vi "Host.vi"() -> ()   [LabVIEW 2019]
uses:
  <vilib>/Analysis/7linalg.llb/Eigenvalue and Vectors Output Option.ctl
  <vilib>/Analysis/baseanly.llb/Matrix Type of Inverse Matrix.ctl
  <vilib>/Analysis/7linalg.llb/Real Generalized Eigenvalues and Vectors.vi
  <vilib>/Analysis/7linalg.llb/Real Cholesky Factorization.vi
  <vilib>/Analysis/baseanly.llb/Full Cholesky Factorization.vi
  <vilib>/Analysis/baseanly.llb/Full Real Matrix Cholesky Factorization.vi
  <vilib>/FPGAPlugInAG/PXIe-7915/niLvFpga_Open_PXIe-7915.vi
  <vilib>/rvi/interface/common/dynamic/niFpgaDynamicAddResources.vi
  <vilib>/Analysis/baseanly.llb/Real Inverse Matrix.vi
  <vilib>/Analysis/Matrix/Numeric/Multiply/Multiply - RM,RM.vi
  <vilib>/Analysis/7linalg.llb/Real Eigenvalues and Vectors.vi
  <vilib>/Analysis/Matrix/Numeric/Add/Add - RM,RM.vi
  <vilib>/Utility/error.llb/Error Cluster From Error Code.vi
  <vilib>/rvi/errors/niLvFpgaAdjustHostInterfaceError.vi
  <vilib>/FPGAPlugInAG/Dynamic/niLvFpga_Run_Dynamic.vi
  <vilib>/FPGAPlugInAG/Dynamic/niLvFpga_Close_Dynamic.vi
  <vilib>/rvi/interface/nirviOpenFPGA/nirviOpenFPGA.xnode
  FPGA Bitfiles/choleskyfpgav1_FPGATarget_Target_zgTmfM5OUWw.lvbitx
  <vilib>/rvi/interface/nirviMethod/nirviMethod.xnode
  <vilib>/rvi/interface/nirviReadWriteControl/nirviReadWriteControl.xnode
  <vilib>/rvi/interface/nirviCloseFPGA/nirviCloseFPGA.xnode
  <vilib>/Analysis/NI_AALPro.lvlib
  <vilib>/Analysis/NI_AALBase.lvlib
  <vilib>/Analysis/Matrix/NI_Matrix.lvlib
  <vilib>/rvi/errors/niLvFpgaMergeErrorWithErrorCode.vi
  <vilib>/FPGAPlugInAG/Dynamic/niLvFpga_ReadFifo_Dynamic.vi
  <vilib>/FPGAPlugInAG/Dynamic/niLvFpga_WriteFifo_Dynamic.vi
  NiFpgaLv.dll
  <vilib>/rvi/interface/Simulation/niFpgaSimulationCallBeginRW.vi
panel:
  out "total time us":u32
  out "T2 tick (ticks)":u32
  out "T5-T4 us":u32
  out "T4-T3 us":u32
  out "T3-T2 us":u32
  out "T2-T1 us":u32
  out "T5 us":u16
  out "T4 us":u16
  out "T3 us":u16
  out "T2 us":u16
  out "T1 us":u16
  out "data output time (ticks)":u32
  out "data input time (ticks)":u32
  out "total time (ticks)":u32
  out "T5 (ticks)":u32
  out "T4 (ticks)":u32
  out "T3 (ticks)":u32
  out "T1 (ticks)":u32
  out "Frequencies":dbl[](array[numeric])
  out "Eigenvalues":cdb[][](array[numeric]) format="%#_4g"
  out "Run Time (ms)":u32 format="%_6f"
  out "Elements Remaining 2":u32
  out "Elements Remaining":u32
  out "K input":dbl[][](array[numeric])
  in  "Method":i32(listbox)
  out "M input":dbl[][](array[numeric])
  # "Takes 56 ms to solve without timed loop"
  # "base"
  # "1087"
  # "2174"
  # "1087"
  # "97"
  # "1087"
  # "1183"
  # "eith timed loops"
  # "AVG. of 13"
  # "AVG. of 289"
  # "AVG. of 289"
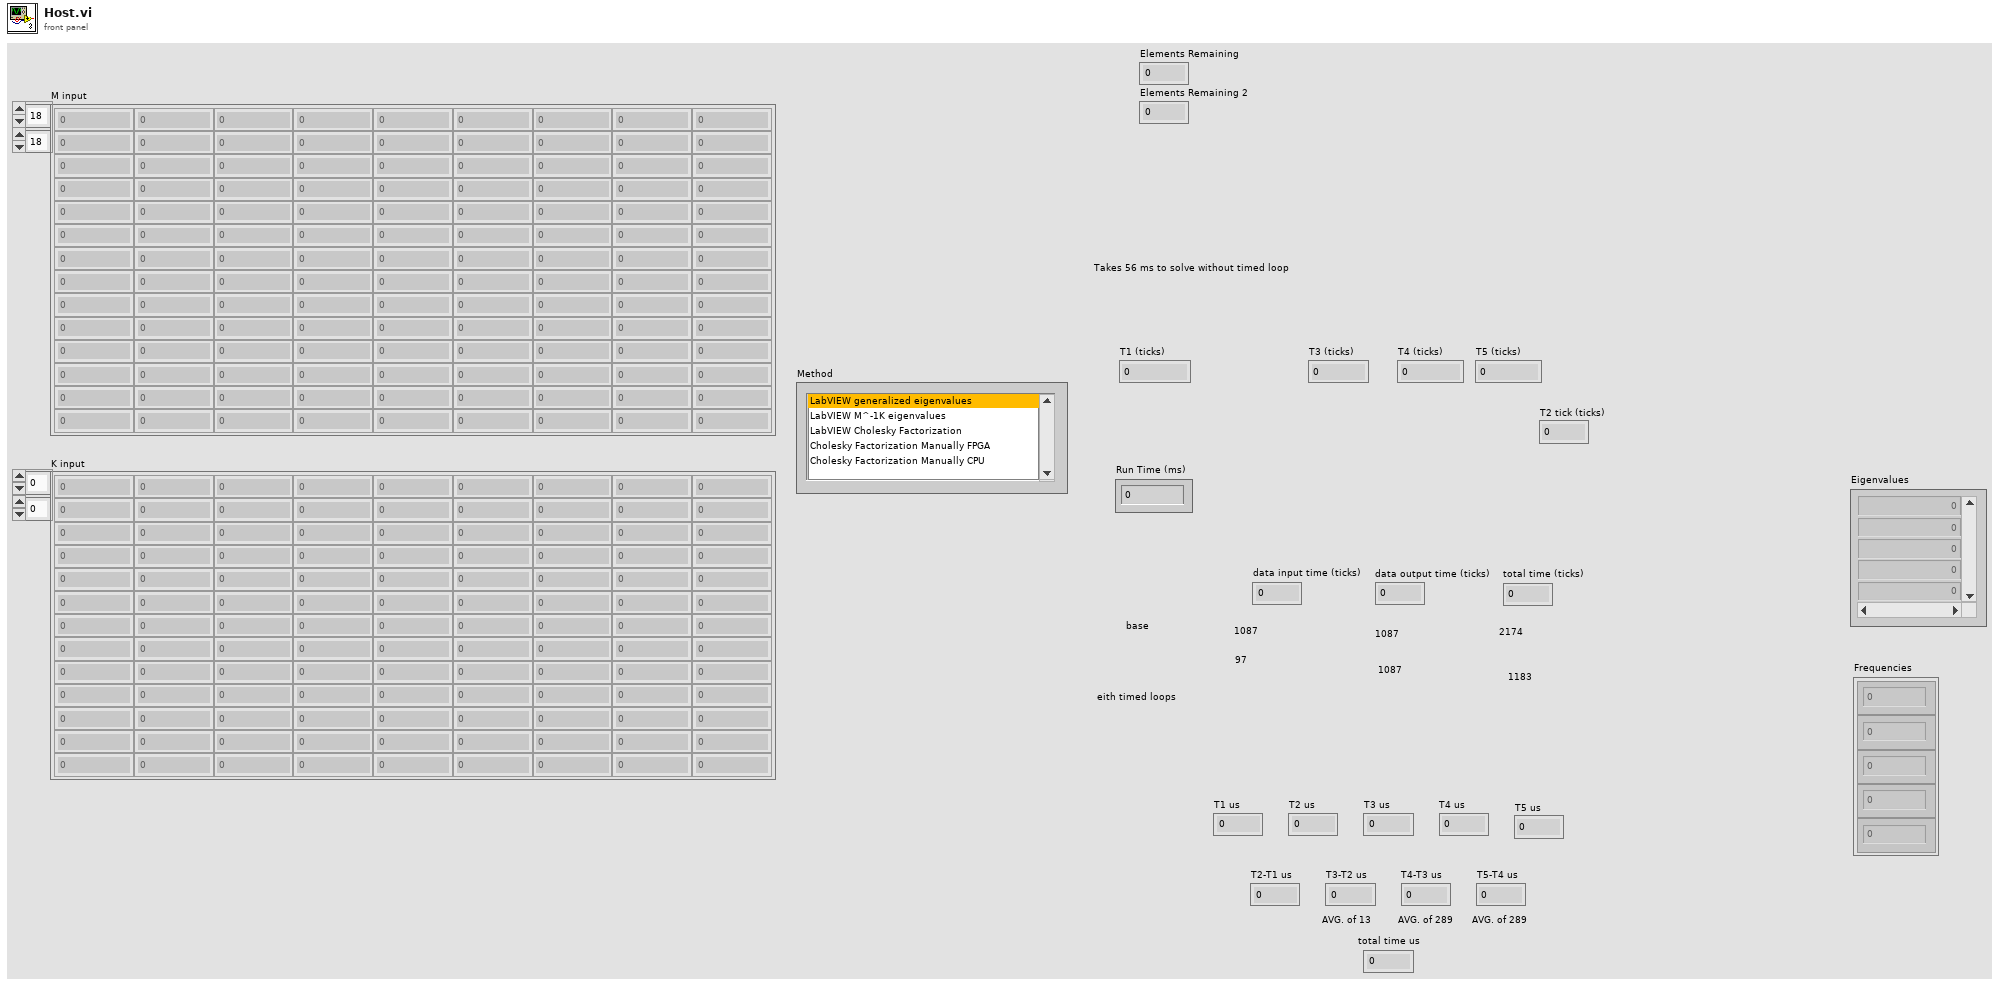
[diagram p1: front panel]
types:
  T1 = typedef "NI_AALBase.lvlib/Matrix Type of Inverse Matrix.ctl" = enum32{"General", "Positive Definite", "Lower Triangular", "Upper Triangular"}
  T2 = typedef "NI_AALPro.lvlib/Eigenvalue and Vectors Output Option.ctl" = i32
  T3 = typedef "NI_Matrix.lvlib/RealMatrix.ctl" = dbl[][]
  T4 = typedef "NI_Matrix.lvlib/ComplexMatrix.ctl" = cdb[][]
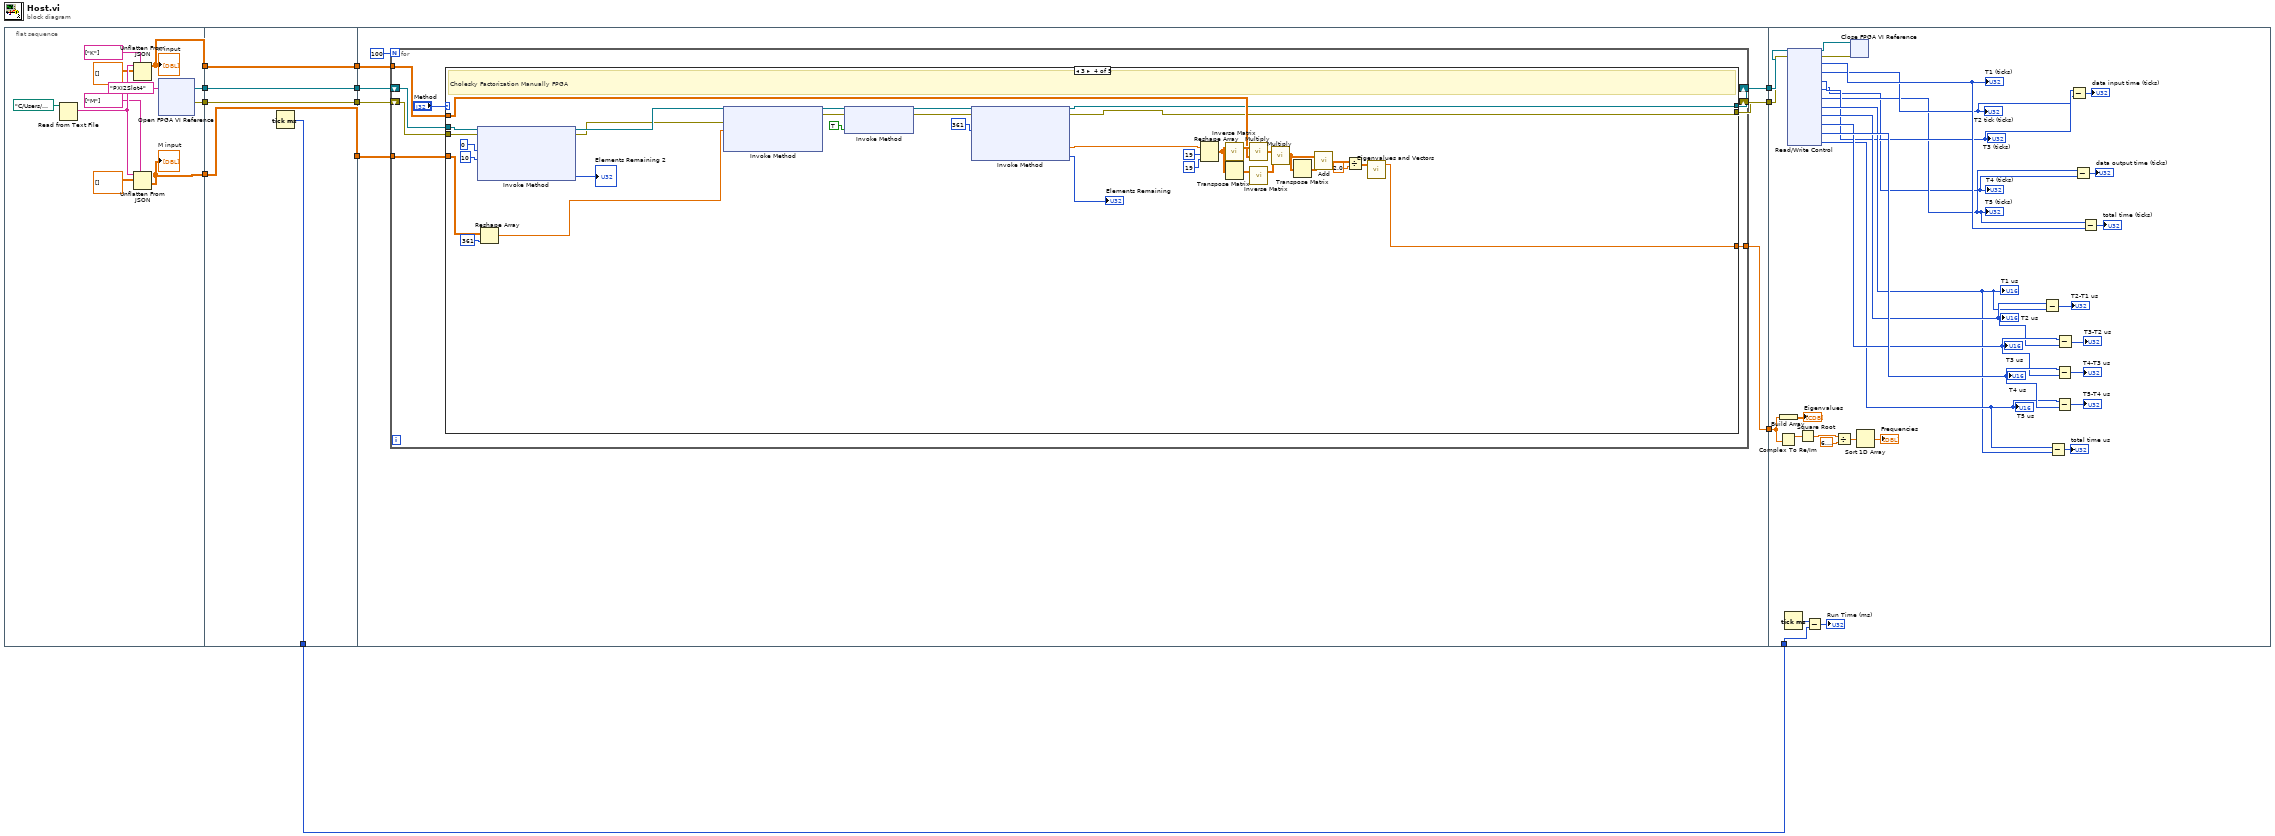
[diagram p0: block diagram]
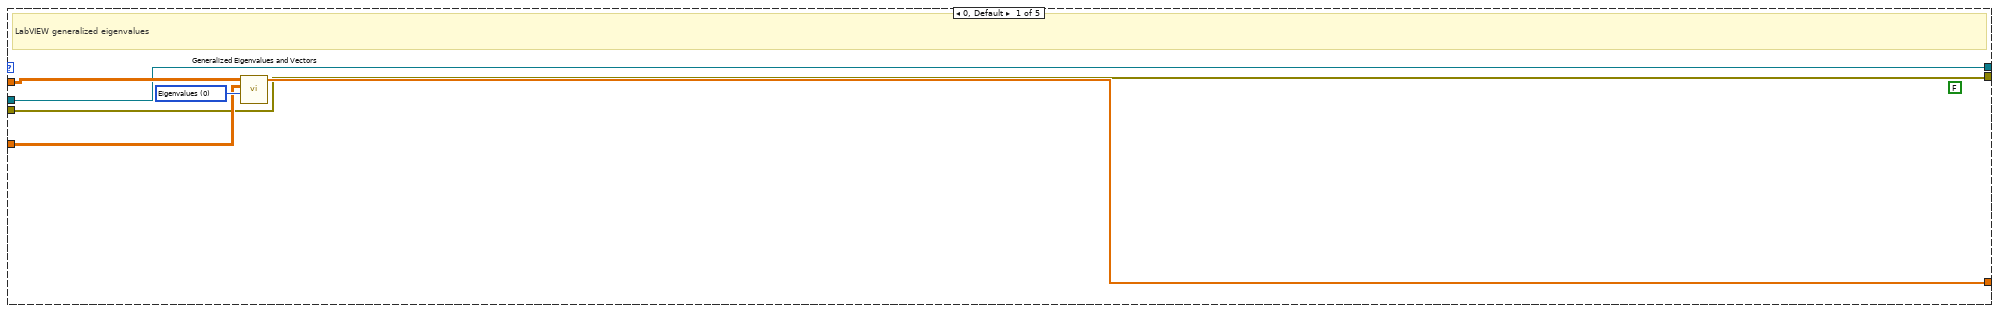
[diagram p2: hidden frame]
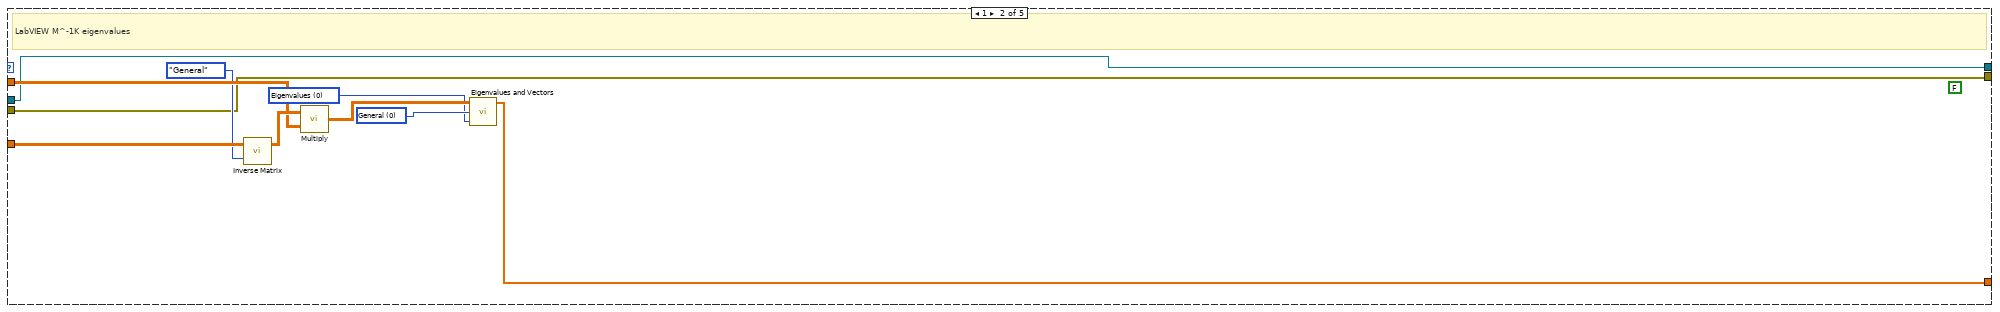
[diagram p3: hidden frame]
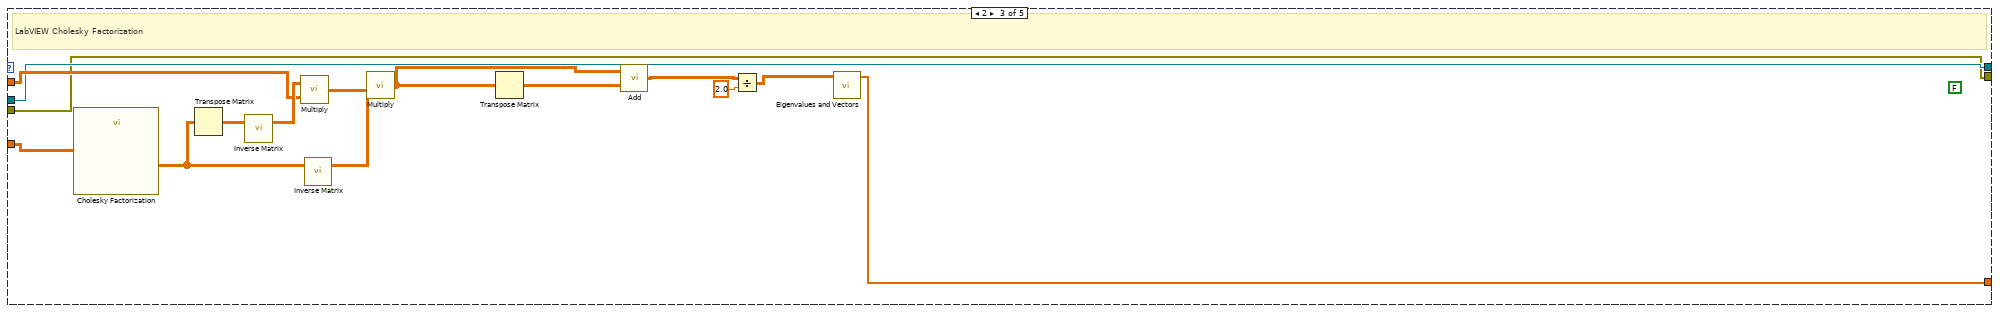
[diagram p4: hidden frame]
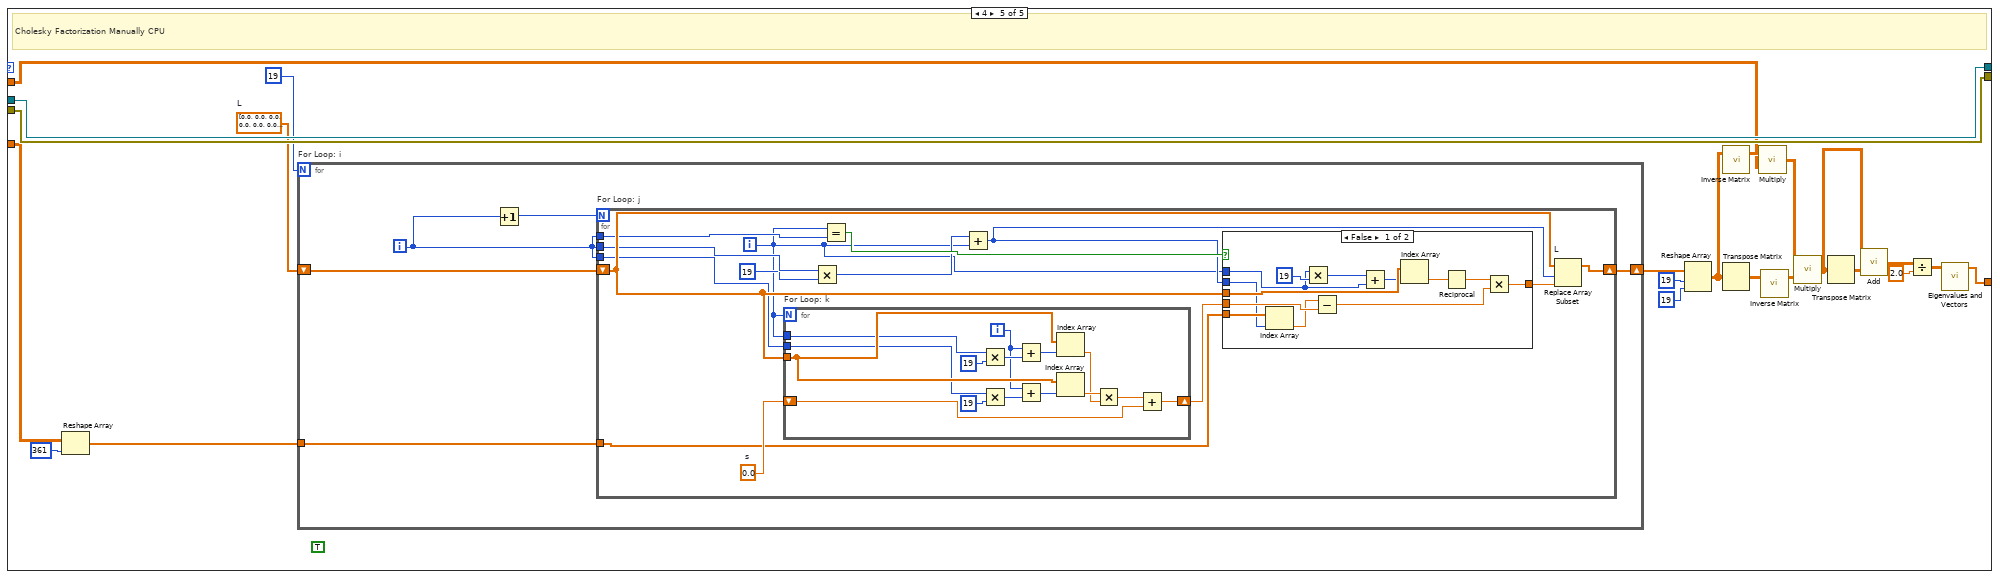
[diagram p5: hidden frame]
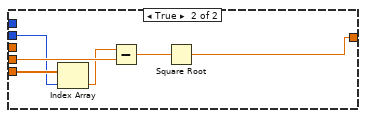
[diagram p6: hidden frame]
diagram:
  n1 = flat-sequence {
    tunnel: [w17] -> w10
    tunnel: [w16] -> w9
    tunnel: [w15] -> w7
    tunnel: [w14] -> w5
    tunnel: [w28] -> w12
    tunnel: [w27] -> w11
    tunnel: [w26] -> w1
    tunnel: w10 -> [w28]
    tunnel: w9 -> [w27]
    tunnel: [w25] -> w8
    tunnel: w7 -> [w25]
    tunnel: [w24] -> w6
    tunnel: w5 -> [w24]
    tunnel: w12 -> [w36]
    tunnel: w11 -> [w35]
    tunnel: w8 -> [w30]
    tunnel: w6 -> [w29]
    tunnel: [w34] -> w4
    tunnel: [w32] -> w3
    tunnel: [w31] -> w2
    tunnel: w4 -> [w208]
    tunnel: w3 -> [w207]
    tunnel: w2 -> [w206]
    tunnel: w1 -> [w205]
    frame #0 {
      n2 = Read from Text File(file (use dialog)=path "C:/Users/PXIe-8880/Documents/AFRL_summer_2019/Cholesky_FPGA/Cholesky_FPGA_V1/data/data.txt") -> (text=w23:string)  [unwired: 3 in, 3 out]
      n3 = Unflatten From JSON(path=string[] ["K"], JSON string=w23, type and defaults=dbl[][] []) -> (value=w16:dbl[][])  [unwired: 4 in, 1 out]
      "K input" <- w16
      n4 = Unflatten From JSON(path=string[] ["M"], JSON string=w23, type and defaults=dbl[][] []) -> (value=w17:dbl[][])  [unwired: 4 in, 1 out]
      "M input" <- w17
      n5 = xnode "Open FPGA VI Reference"("resource name"=tag "PXI2Slot4") -> ("FPGA VI Reference Out"=w15:refnum<k20>, "error out"=w14:errorcluster)  [unwired: 1 in]
    }
    frame #1 {
      n6 = Tick Count (ms)() -> (millisecond timer value=w26:u32)
    }
    frame #2 {
      n7 = for {
        N: 100 -> [_]
        tunnel: w36 -> [w44]
        tunnel: w35 -> [w43]
        tunnel: [w40] -> w34
        shift-right: [w42] -> w32
        shift-left: w30 -> [w38]
        shift-right: [w41] -> w31
        shift-left: w29 -> [w37]
        n8 = case shown="3" "Method" {
          tunnel: [w49 w56 w69 w94 w110] -> w40
          tunnel: w44 -> [w48 w55 w75 w109 w111]
          tunnel: w43 -> [w47 w54 w71 w95 w112]
          tunnel: w38 -> [w46 w52 w62 w84 w131]
          tunnel: [w46 w52 w62 w88 w131] -> w42
          tunnel: w37 -> [w45 w51 w61 w83 w130]
          tunnel: [w45 w51 w61 w89 w130] -> w41
          frame 0, Default {
            (unwired) FALSE
            w50 = T2 0 items=["Eigenvalues", "Eigenvalues & Vectors"] ("output option")
            # "LabVIEW generalized eigenvalues"
            n9 = call-poly <vilib>:"Generalized Eigenvalues and Vectors.vi"("output option"=w50, "B"=w48, "A"=w47) -> ("Eigenvalues"=w49:cdb[])  [unwired: 3 in, 2 out]
          }
          frame 1 {
            (unwired) FALSE
            w57 = T2 0 items=["Eigenvalues", "Eigenvalues & Vectors"] ("output option")
            w58 = 0 items=["General", "Symmetric"] ("matrix type")
            # "LabVIEW M^-1K eigenvalues"
            n10 = call-poly <vilib>:"Inverse Matrix.vi"("matrix type"=Matrix_Type_of_Inverse_Matrix."General", "Input Matrix"=w55) -> ("Inverse Matrix"=w59:T3)  [unwired: 1 out]
            n11 = call-poly <vilib>:"Multiply.vi"("Real Matrix B"=w54, "Real Matrix A"=w59) -> ("A * B"=w60:T3)
            n12 = call-poly <vilib>:"Eigenvalues and Vectors.vi"("output option"=w57, "matrix type"=w58, "Input Matrix"=w60) -> ("Eigenvalues"=w56:cdb[])  [unwired: 2 out]
          }
          frame 2 {
            (unwired) FALSE
            # "LabVIEW Cholesky Factorization"
            n13 = call-poly <vilib>:"Cholesky Factorization.vi"("A"=w75) -> ("Cholesky"=w73:T3)  [unwired: 1 out]
            n14 = Transpose Matrix(1:w73) -> (0:w74:T3)
            n15 = call-poly <vilib>:"Inverse Matrix.vi"("Input Matrix"=w74) -> ("Inverse Matrix"=w72:T3)  [unwired: 1 in, 1 out]
            n16 = call-poly <vilib>:"Multiply.vi"("Real Matrix B"=w71, "Real Matrix A"=w72) -> ("A * B"=w68:T3)
            n17 = call-poly <vilib>:"Inverse Matrix.vi"("Input Matrix"=w73) -> ("Inverse Matrix"=w70:T3)  [unwired: 1 in, 1 out]
            n18 = call-poly <vilib>:"Multiply.vi"("Real Matrix B"=w70, "Real Matrix A"=w68) -> ("A * B"=w67:T3)
            n19 = Transpose Matrix(1:w67) -> (0:w66:T3)
            n20 = call-poly <vilib>:"Add.vi"("Real Matrix B"=w66, "Real Matrix A"=w67) -> ("A + B"=w64:T3)
            n21 = Divide(x=w64, y=2.0) -> (x/y=w63:T3)
            n22 = call-poly <vilib>:"Eigenvalues and Vectors.vi"("Input Matrix"=w63) -> ("Eigenvalues"=w69:cdb[])  [unwired: 2 in, 2 out]
          }
          frame 3 {
            # "Cholesky Factorization Manually FPGA"
            n23 = xnode "Invoke Method"("FPGA VI Reference In"=w84, "error in"=w83, "Number of Elements"=u32 0, "Timeout (ms)"=10) -> ("FPGA VI Reference Out"=w82:refnum<k20>, "error out"=w81:errorcluster, "Elements Remaining"=→"Elements Remaining 2":u32)  [unwired: 1 out]
            n24 = Reshape Array(w109, 361 ("dimension size")) -> (w78:dbl[])
            n25 = xnode "Invoke Method"("FPGA VI Reference In"=w82, "error in"=w81, "Data"=w78) -> ("FPGA VI Reference Out"=w93:refnum<k20>, "error out"=w92:errorcluster)  [unwired: 1 in, 1 out]
            n26 = xnode "Invoke Method"("FPGA VI Reference In"=w93, "error in"=w92, "Wait Until Done (F)"=TRUE) -> ("FPGA VI Reference Out"=w91:refnum<k20>, "error out"=w90:errorcluster)
            n27 = xnode "Invoke Method"("FPGA VI Reference In"=w91, "error in"=w90, "Number of Elements"=u32 361) -> ("FPGA VI Reference Out"=w88:refnum<k20>, "error out"=w89:errorcluster, "Data"=w77:sgl[], "Elements Remaining"=→"Elements Remaining":u32)  [unwired: 1 in]
            n28 = Reshape Array(w77, 19 ("dimension size"), 19 ("dimension size")) -> (w76:sgl[][])
            n29 = call-poly <vilib>:"Inverse Matrix.vi"("Input Matrix"=w76) -> ("Inverse Matrix"=w104:T3)  [unwired: 1 in, 1 out]
            n30 = Transpose Matrix(1:w76) -> (0:w96:dbl[][])
            n31 = call-poly <vilib>:"Multiply.vi"("Real Matrix B"=w95, "Real Matrix A"=w104) -> ("A * B"=w102:T3)
            n32 = call-poly <vilib>:"Inverse Matrix.vi"("Input Matrix"=w96) -> ("Inverse Matrix"=w103:T3)  [unwired: 1 in, 1 out]
            n33 = call-poly <vilib>:"Multiply.vi"("Real Matrix B"=w103, "Real Matrix A"=w102) -> ("A * B"=w101:T3)
            n34 = Transpose Matrix(1:w101) -> (0:w100:T3)
            n35 = call-poly <vilib>:"Add.vi"("Real Matrix B"=w100, "Real Matrix A"=w101) -> ("A + B"=w98:T3)
            n36 = Divide(x=w98, y=2.0) -> (x/y=w97:T3)
            n37 = call-poly <vilib>:"Eigenvalues and Vectors.vi"("Input Matrix"=w97) -> ("Eigenvalues"=w94:cdb[])  [unwired: 2 in, 2 out]
          }
          frame 4 {
            w129 = sgl[] [0.0, 0.0, 0.0, 0.0, 0.0, 0.0, 0.0, 0.0, 0.0, 0.0, 0.0, 0.0, 0.0, 0.0, 0.0, 0.0, 0.0, 0.0, 0.0, 0.0, 0.0, 0.0, 0.0, 0.0, 0.0, 0.0, 0.0, 0.0, 0.0, 0.0, 0.0, 0.0, 0.0, 0.0, 0.0, 0.0, 0.0, 0.0, 0.0, 0.0, 0.0, 0.0, 0.0, 0.0, 0.0, 0.0, 0.0, 0.0, 0.0, 0.0, 0.0, 0.0, 0.0, 0.0, 0.0, 0.0, 0.0, 0.0, 0.0, 0.0, 0.0, 0.0, 0.0, 0.0, 0.0, 0.0, 0.0, 0.0, 0.0, 0.0, 0.0, 0.0, 0.0, 0.0, 0.0, 0.0, 0.0, 0.0, 0.0, 0.0, 0.0, 0.0, 0.0, 0.0, 0.0, 0.0, 0.0, 0.0, 0.0, 0.0, 0.0, 0.0, 0.0, 0.0, 0.0, 0.0, 0.0, 0.0, 0.0, 0.0, 0.0, 0.0, 0.0, 0.0, 0.0, 0.0, 0.0, 0.0, 0.0, 0.0, 0.0, 0.0, 0.0, 0.0, 0.0, 0.0, 0.0, 0.0, 0.0, 0.0, 0.0, 0.0, 0.0, 0.0, 0.0, 0.0, 0.0, 0.0, 0.0, 0.0, 0.0, 0.0, 0.0, 0.0, 0.0, 0.0, 0.0, 0.0, 0.0, 0.0, 0.0, 0.0, 0.0, 0.0, 0.0, 0.0, 0.0, 0.0, 0.0, 0.0, 0.0, 0.0, 0.0, 0.0, 0.0, 0.0, 0.0, 0.0, 0.0, 0.0, 0.0, 0.0, 0.0, 0.0, 0.0, 0.0, 0.0, 0.0, 0.0, 0.0, 0.0, 0.0, 0.0, 0.0, 0.0, 0.0, 0.0, 0.0, 0.0, 0.0, 0.0, 0.0, 0.0, 0.0, 0.0, 0.0, 0.0, 0.0, 0.0, 0.0, 0.0, 0.0, 0.0, 0.0, 0.0, 0.0, 0.0, 0.0, 0.0, 0.0, 0.0, 0.0, 0.0, 0.0, 0.0, 0.0, 0.0, 0.0, 0.0, 0.0, 0.0, 0.0, 0.0, 0.0, 0.0, 0.0, 0.0, 0.0, 0.0, 0.0, 0.0, 0.0, 0.0, 0.0, 0.0, 0.0, 0.0, 0.0, 0.0, 0.0, 0.0, 0.0, 0.0, 0.0, 0.0, 0.0, 0.0, 0.0, 0.0, 0.0, 0.0, 0.0, 0.0, 0.0, 0.0, 0.0, 0.0, 0.0, 0.0, 0.0, 0.0, 0.0, 0.0, 0.0, 0.0, 0.0, 0.0, 0.0, 0.0, 0.0, 0.0, 0.0, 0.0, 0.0, 0.0, 0.0, 0.0, 0.0, 0.0, 0.0, 0.0, 0.0, 0.0, 0.0, 0.0, 0.0, 0.0, 0.0, 0.0, 0.0, 0.0, 0.0, 0.0, 0.0, 0.0, 0.0, 0.0, 0.0, 0.0, 0.0, 0.0, 0.0, 0.0, 0.0, 0.0, 0.0, 0.0, 0.0, 0.0, 0.0, 0.0, 0.0, 0.0, 0.0, 0.0, 0.0, 0.0, 0.0, 0.0, 0.0, 0.0, 0.0, 0.0, 0.0, 0.0, 0.0, 0.0, 0.0, 0.0, 0.0, 0.0, 0.0, 0.0, 0.0, 0.0, 0.0, 0.0, 0.0, 0.0, 0.0, 0.0, 0.0, 0.0, 0.0, 0.0, 0.0, 0.0, 0.0, 0.0, 0.0, 0.0, 0.0, 0.0, 0.0, 0.0, 0.0, 0.0, 0.0, 0.0, 0.0, 0.0, 0.0, 0.0, 0.0, 0.0, 0.0, 0.0, 0.0, 0.0, 0.0, 0.0]  # L
            (unwired) TRUE
            # "Cholesky Factorization Manually CPU"
            n38 = Reshape Array(w111, 361 ("dimension size")) -> (w126:dbl[])
            n39 = for "For Loop: i" {
              N: 19 -> [_]
              shift-right: [w134] -> w114
              shift-left: w129 -> [w136]
              tunnel: w126 -> [w133]
              i -> [w132]
              n40 = Increment(x=w132) -> (x+1=w135:i32)
              n41 = for "For Loop: j" {
                N: w135 -> [_]
                tunnel: w132 -> [w144]
                shift-right: [w146] -> w134
                shift-left: w136 -> [w145]
                tunnel: w132 -> [w143]
                tunnel: w133 -> [w140]
                tunnel: w132 -> [w138]
                i -> [w137]
                w149 = sgl 0.0  # s
                n42 = for "For Loop: k" {
                  N: w137 -> [_]
                  tunnel: w145 -> [w183]
                  shift-right: [w179] -> w148
                  shift-left: w149 -> [w180]
                  tunnel: w138 -> [w178]
                  tunnel: w137 -> [w171]
                  i -> [w170]
                  n43 = Multiply(x=w171, y=19) -> (x*y=w173:i32)
                  n44 = Multiply(x=w178, y=19) -> (x*y=w176:i32)
                  n45 = Add(x=w170, y=w173) -> (x+y=w172:i32)
                  n46 = Add(x=w170, y=w176) -> (x+y=w175:i32)
                  n47 = Index Array(array=w183, index=w172) -> (element=w182:sgl)
                  n48 = Index Array(array=w183, index=w175) -> (element=w184:sgl)
                  n49 = Multiply(x=w184, y=w182) -> (x*y=w181:sgl)
                  n50 = Add(x=w181, y=w180) -> (x+y=w179:sgl)
                }
                n51 = Multiply(x=w143, y=19) -> (x*y=w141:i32)
                n52 = Equal?(x=w137, y=w144) -> (x = y?=w150:bool)
                n53 = Add(x=w141, y=w137) -> (x+y=w139:i32)
                n54 = case shown="False" w150 {
                  tunnel: w148 -> [w161 w169]
                  tunnel: [w160 w167] -> w147
                  tunnel: w145 -> [w163 _]
                  tunnel: w140 -> [w157 w166]
                  tunnel: w139 -> [w156 w165]
                  tunnel: w137 -> [w152 _]
                  frame False {
                    n55 = Index Array(array=w157, index=w156) -> (element=w155:dbl)
                    n56 = Multiply(x=w152, y=19) -> (x*y=w153:i32)
                    n57 = Subtract(x=w155, y=w161) -> (x-y=w158:dbl)
                    n58 = Add(x=w153, y=w152) -> (x+y=w151:i32)
                    n59 = Index Array(array=w163, index=w151) -> (element=w162:sgl)
                    n60 = Reciprocal(x=w162) -> (1/x=w159:sgl)
                    n61 = Multiply(x=w159, y=w158) -> (x*y=w160:dbl)
                  }
                  frame True {
                    n62 = Index Array(array=w166, index=w165) -> (element=w164:dbl)
                    n63 = Subtract(x=w164, y=w169) -> (x-y=w168:dbl)
                    n64 = Square Root(x=w168) -> (sqrt(x)=w167:dbl)
                  }
                }
                n65 = Replace Array Subset "L"(array=w145, new element=w147, index=w139) -> (w146:sgl[])
              }
            }
            n66 = Reshape Array(w114, 19 ("dimension size"), 19 ("dimension size")) -> (w113:sgl[][])
            n67 = call-poly <vilib>:"Inverse Matrix.vi"("Input Matrix"=w113) -> ("Inverse Matrix"=w123:T3)  [unwired: 1 in, 1 out]
            n68 = Transpose Matrix(1:w113) -> (0:w115:dbl[][])
            n69 = call-poly <vilib>:"Multiply.vi"("Real Matrix B"=w112, "Real Matrix A"=w123) -> ("A * B"=w121:T3)
            n70 = call-poly <vilib>:"Inverse Matrix.vi"("Input Matrix"=w115) -> ("Inverse Matrix"=w122:T3)  [unwired: 1 in, 1 out]
            n71 = call-poly <vilib>:"Multiply.vi"("Real Matrix B"=w122, "Real Matrix A"=w121) -> ("A * B"=w120:T3)
            n72 = Transpose Matrix(1:w120) -> (0:w119:T3)
            n73 = call-poly <vilib>:"Add.vi"("Real Matrix B"=w119, "Real Matrix A"=w120) -> ("A + B"=w117:T3)
            n74 = Divide(x=w117, y=2.0) -> (x/y=w116:T3)
            n75 = call-poly <vilib>:"Eigenvalues and Vectors.vi"("Input Matrix"=w116) -> ("Eigenvalues"=w110:cdb[])  [unwired: 2 in, 2 out]
          }
        }
      }
    }
    frame #3 {
      n76 = Build Array(w208) -> (→"Eigenvalues":T4)
      n77 = Complex To Re/Im ("Complex To Cartesian.vi")(x + iy=w208) -> (x=w214:dbl[])  [unwired: 1 out]
      n78 = Tick Count (ms)() -> (millisecond timer value=w204:u32)
      n79 = xnode "Read/Write Control"("FPGA VI Reference In"=w207, "error in"=w206) -> ("FPGA VI Reference Out"=w210:refnum<k20>, "error out"=w209:errorcluster, "T1 tick"=w192:u32, "T2 tick"=w187:u32, "T3 tick"=w188:u32, "T4 tick"=w185:u32, "T5 ticks"=w186:u32, "T1 us"=w189:u16, "T2 us"=w193:u16, "T3 us"=w194:u16, "T4 us"=w195:u16, "T5 us"=w190:u16)
      "T1 (ticks)" <- w192
      "T3 (ticks)" <- w188
      "T4 (ticks)" <- w185
      "T5 (ticks)" <- w186
      "T1 us" <- w189
      "T2 us" <- w193
      "T3 us" <- w194
      "T4 us" <- w195
      "T5 us" <- w190
      "T2 tick (ticks)" <- w187
      n80 = Square Root ("Square Root.vi")(x=w214) -> (sqrt(x)=w215:dbl[])
      n81 = Subtract(x=w204, y=w205) -> (x-y=→"Run Time (ms)":u32)
      n82 = Divide(x=w215, y=6.283185307179586) -> (x/y=w216:dbl[])
      n83 = xnode "Close FPGA VI Reference"("FPGA VI Reference In"=w210, "error in"=w209) -> ()  [unwired: 1 out]
      n84 = Sort 1D Array(array=w216) -> (sorted array=→"Frequencies":dbl[])
      n85 = Subtract(x=w193, y=w189) -> (x-y=→"T2-T1 us":u16)
      n86 = Subtract(x=w190, y=w189) -> (x-y=→"total time us":u16)
      n87 = Subtract(x=w195, y=w194) -> (x-y=→"T4-T3 us":u16)
      n88 = Subtract(x=w190, y=w195) -> (x-y=→"T5-T4 us":u16)
      n89 = Subtract(x=w194, y=w193) -> (x-y=→"T3-T2 us":u16)
      n90 = Subtract(x=w188, y=w187) -> (x-y=→"data input time (ticks)":u32)
      n91 = Subtract(x=w186, y=w185) -> (x-y=→"data output time (ticks)":u32)
      n92 = Subtract(x=w186, y=w192) -> (x-y=→"total time (ticks)":u32)
    }
  }
